vi "Main.vi"() -> ()   [LabVIEW 2015] (continued)
  out "Sigma":dbl[](array[numeric])
  out "Last Zernike":dbl[](array[numeric])
  in  "Stop AO Algorithm":bool
  in  "Step Size":dbl=0.05
  out "Metric Value":dbl(graph)=0.00227571952127783
  out "Optimal Zernike":dbl[](array[numeric])
  out "Quadratic Calc":bool
  out "Optimal Z Idx":i32
  in  "Note":string="Cou6_200x200_5mW_1580nm_step0.01"
  # "Up"
  # "Right"
  # "Left"
  # "Down"
  # "Standard Lifetimes (s):\nCoumarin 6 MeOH - 2.3E-9\nCoumarin 6 EtOH - 2.41E-9\nFluorescein NaOH - 4.0E-9\nRhodamine B H2O - 1.7E-9"
  # "V_IF (0 or -2pi)"
  # "(Shutter On)"
  # "(Shutter Off)"
  # "V_IF (0.5pi or -1.5pi)"
  # "V_IF (pi or -pi)"
  # "V_IF (1.5pi or -0.5pi)"
  # "Pixel width calibration:\n1. Move the cursor to a feature pixel that you can recognize\n2. Click \"Record X1\" to record the X coordinate\n\n \n3. Use \"X-\" or \"X+\" with \"XY Step\" of 30 um to move the image horizentally by 30 um\n4. Move the cursor to the same feature pixel\n5. Click \"Record X2\" to record the X coordinate again\n\n\n6. Click \"Pixel Width\" to calculate the pixel width (um/px)\n7. Input your desired pixel width (um/px) and the cooresponding \"XY Factor (1/V)\" will be calculated"
  # "Based on \"Desired Pixel Wdith (um)\""
  # "Going inside the sample (Z increase)"
  # "Z4\nAst45"
  # "Z5\nDef"
  # "Z6\nAst0"
  # "Z7\nTreY"
  # "Z8\nComX"
  # "Z9\nComY"
  # "Z10\nTreX"
  # "Z11\nTetY"
  # "Z12\nSAstY"
  # "Z13\nSAb3"
  # "Z14\nSAstX"
  # "Z15\nTetX"
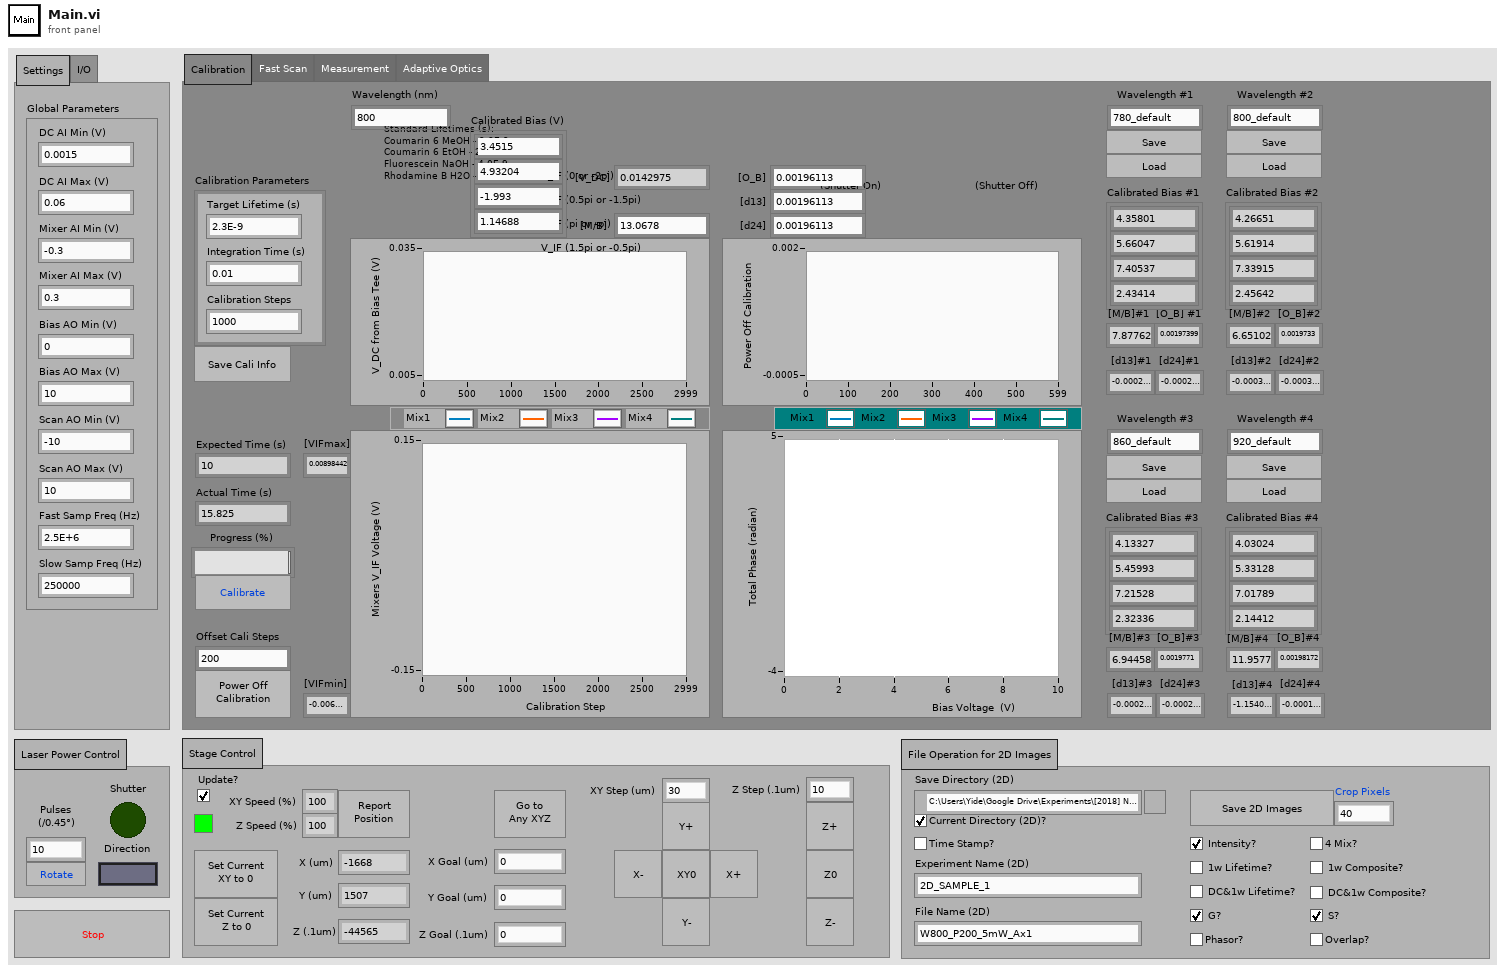
[diagram p1: front panel]
types:
  T1 = cluster{"DC AI Min (V)":dbl, "DC AI Max (V)":dbl, "Mixer AI Min (V)":dbl, "Mixer AI Max (V)":dbl, "Bias AO Min (V)":dbl, "Bias AO Max (V)":dbl, "Scan AO Min (V)":dbl, "Scan AO Max (V)":dbl, "Fast Samp Freq (Hz)":dbl, "Slow Samp Freq (Hz)":dbl}
  T2 = enum32{"Calibration", "Fast Scan", "Measurement", "Adaptive Optics"}
  T3 = cluster{"Target Lifetime (s)":dbl, "Integration Time (s)":dbl, "Calibration Steps":dbl}
  T4 = cluster{"Pixel Dwell Time (s)":dbl, "Pixel Size":dbl, "X Min (V)":dbl, "X Max (V)":dbl, "Y Min (V)":dbl, "Y Max (V)":dbl, "XY Factor (1/V)":dbl}
  T5 = enum16{"Nikon 40X NA 0.8 WD=3.5mm", "Olympus 25X NA 1.05 WD=2mm"}
  T6 = enum32{"Process", "Results", "Phasors", "Z-Stack", "Time-Lapse", "GSOS Process", "GSOS Results"}
  T7 = cluster{"X Values":dbl[], "Histogram: h(x)":i32[]}
  T8 = enum16{"fire", "rainbow", "gray", "inverse gray", "ice", "original"}
  T9 = cluster{bool[], dbl[], cluster{dbl, dbl}[], u32[]}
  T10 = enum16{"Intensity 3D", "1w Lifetime 3D", "DC&1w Lifetime 3D", "1w Composite 3D", "DC&1w Composite 3D", "Phasor 3D", "Overlap 3D"}
  T11 = enum16{"Mean Pixel Value", "Normalized Variance", "Mean Squared Pixel Value"}
  T12 = cluster{"Mixer AI Channel(s)":tag, "DC AI Channel(s)":tag, "Bias AO Channel(s) ":tag, "Scan AO Channel(s)":tag}
  T13 = enum32{"Calibration", "Fast Scan", "Measurement"}
  T14 = cluster{"DC AI task out":refnum<k21>, "Mixer AI task out":refnum<k21>, "Bias AO task out":refnum<k21>, "Scan AO task out":refnum<k21>}
  T15 = typedef "NI_LVConfig.lvlib/Config Data RefNum.ctl" = refnum<k1>
  T16 = typedef "LVBoundsTypeDef.ctl" = cluster{"Width":u32, "Height":u32}
  T17 = typedef "lveventtype.ctl" = enum32{"Null", "Timeout", "Annotation Menu Selection", "Annotation Menu Selection?", "App Instance Close", "App Instance Close?", "Autoscale Range Change", "Bookmark Info Change", "Cell Edit", "Cell Edit?", "Cursor Grab", "Cursor Grab?", "Cursor Menu Selection", "Cursor Menu Selection?", "Cursor Move", "Cursor Release", "Data Change", "Direction Change", "Display State Change", "Drag Ended", "Drag Enter", "Drag Leave", "Drag Over", "Drag Source Update", "Drag Starting", "Drag Starting?", "Drop", "Exec State Change", "Key Down", "Key Down?", "Key Repeat", "Key Repeat?", "Key Up", "Listbox Double Click", "Menu Activation?", "Menu Selection (App)", "Menu Selection? (App)", "Menu Selection (User)", "Mouse Down", "Mouse Down?", "Mouse Enter", "Mouse Leave", "Mouse Move", "Mouse Up", "Mouse Wheel", "NI Security User Change (App)", "Pane Size", "Panel Close", "Panel Close?", "Panel Resize", "Plot Attribute Change", "Scale Range Change", "Shortcut Menu Activation?", "Shortcut Menu Selection (App)", "Shortcut Menu Selection? (App)", "Shortcut Menu Selection (User)", "Tree Double Click", "Tree Drag", "Tree Drag?", "Tree Drop", "Tree Drop?", "Tree Item Close", "Tree Item Close?", "Tree Item Open", "Tree Item Open?", "User Event", "Value Change"}
  T18 = typedef "LVRectTypeDef.ctl" = cluster{"Left":i16, "Top":i16, "Right":i16, "Bottom":i16}
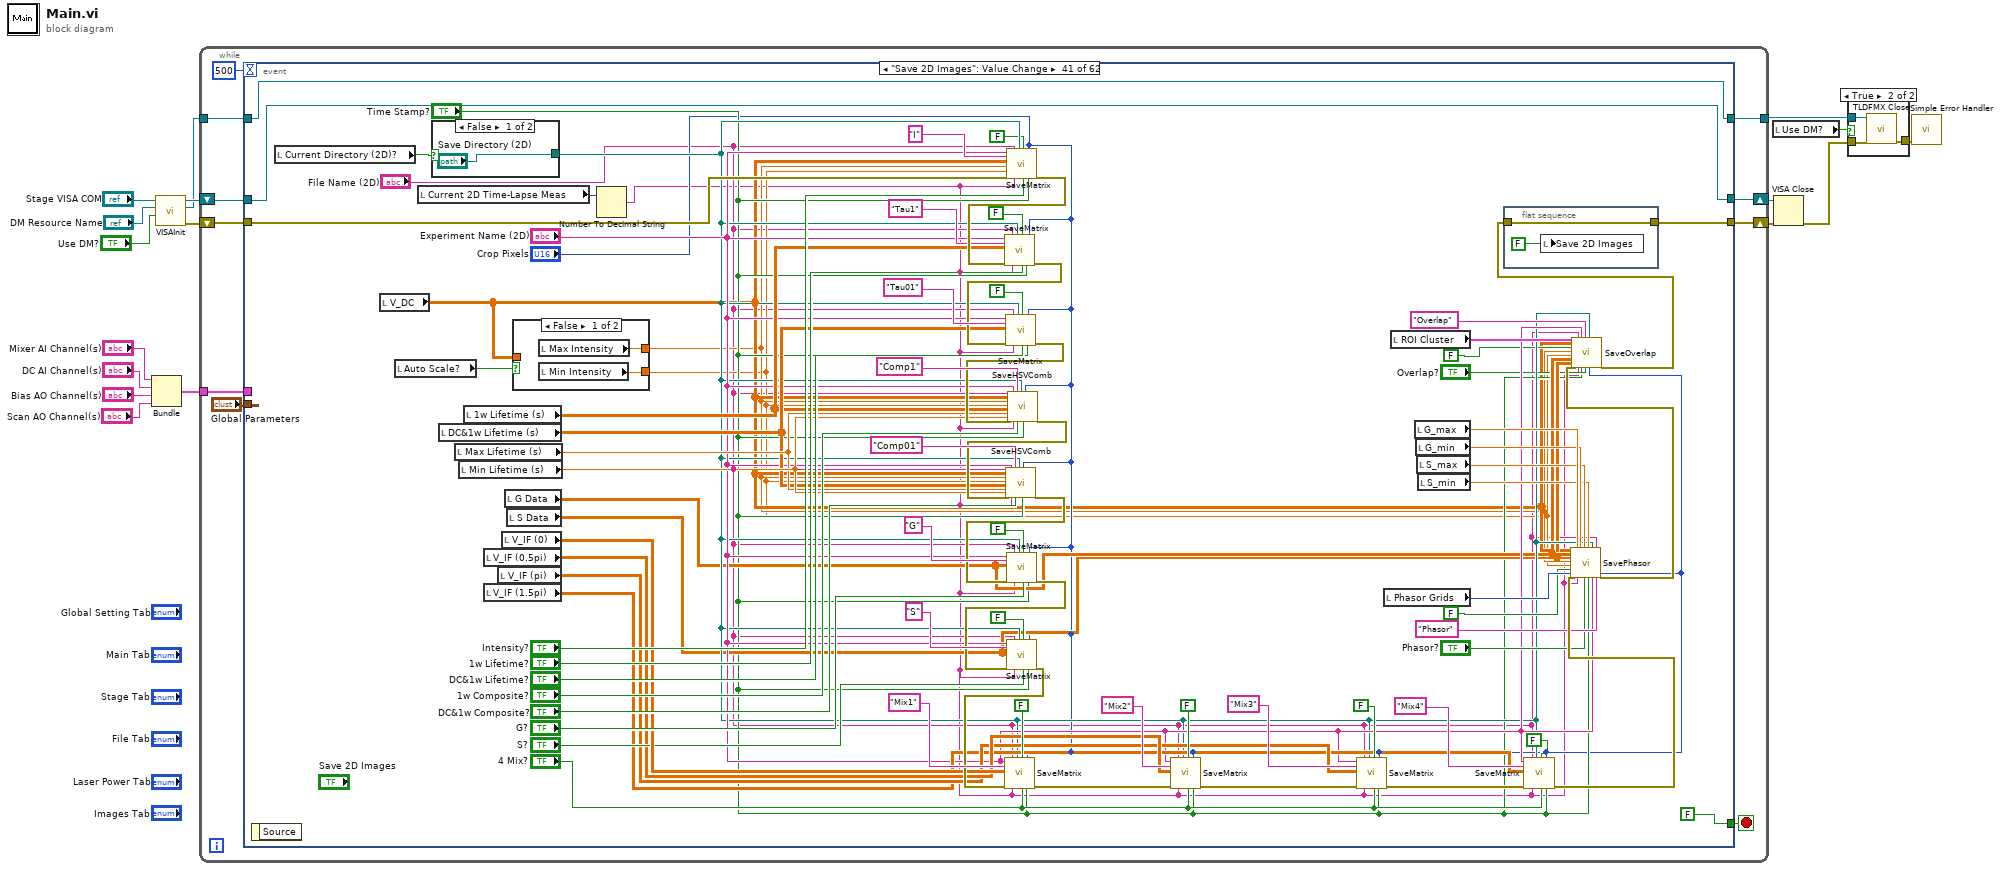
[diagram p0: block diagram]
diagram:
  n1 = Bundle("Mixer AI Channel(s)"="Mixer AI Channel(s)", "DC AI Channel(s)"="DC AI Channel(s)", "Bias AO Channel(s)"="Bias AO Channel(s)", "Scan AO Channel(s)"="Scan AO Channel(s)") -> (w13:T12)  [unwired: 1 in]
  n2 = call "VISAInit.vi"("Use DM?"="Use DM?", "DM Resource Name"="DM Resource Name", "Stage Resource Name"="Stage VISA COM") -> ("error out"=w12:errorcluster, "DM Handle"=w8:refnum<visa-resource-name>, "Stage Resource"=w11:refnum<visa-resource-name>)  [unwired: 6 in]
  n3 = while {
    shift-right: [w22] -> w17
    shift-left: w11 -> [w27]
    shift-right: [w21] -> w16
    shift-left: w12 -> [w26]
    tunnel: w13 -> [w25]
    tunnel: w8 -> [w20]
    tunnel: [w19] -> w5
    stop <- w24 stop-if-true
    n4 = event shown="[40] \"Save 2D Images\": Value Change" {
      selector: _ -> [_ _ _ _ _ _ _ _ _ _ _ _ _ _ _ _ _ _ _ _ _ _ _ _ _ _ _ _ _ _ _ _ _ _ _ _ _ _ _ _ _ _ _ _ _ _ _ _ _ _ _ _ _ _ _ _ _ _ _ _ _ _]
      dyn-events: _ -> [_ _ _ _ _ _ _ _ _ _ _ _ _ _ _ _ _ _ _ _ _ _ _ _ _ _ _ _ _ _ _ _ _ _ _ _ _ _ _ _ _ _ _ _ _ _ _ _ _ _ _ _ _ _ _ _ _ _ _ _ _ _]
      timeout: 500 -> [_ _ _ _ _ _ _ _ _ _ _ _ _ _ _ _ _ _ _ _ _ _ _ _ _ _ _ _ _ _ _ _ _ _ _ _ _ _ _ _ _ _ _ _ _ _ _ _ _ _ _ _ _ _ _ _ _ _ _ _ _ _]
      tunnel: [FALSE ("Shutter") FALSE ("Shutter") FALSE ("Shutter") FALSE ("Shutter") FALSE ("Shutter") FALSE ("Shutter") FALSE ("Shutter") FALSE ("Shutter") FALSE ("Shutter") FALSE ("Shutter") FALSE ("Shutter") FALSE ("Shutter") FALSE ("Shutter") FALSE ("Shutter") FALSE ("Shutter") _ FALSE ("Shutter") _ _ _ _ FALSE ("Shutter") _ FALSE ("Shutter") FALSE ("Shutter") FALSE ("Shutter") FALSE ("Shutter") FALSE ("Shutter") FALSE ("Shutter") FALSE ("Shutter") FALSE ("Shutter") FALSE ("Shutter") FALSE ("Shutter") FALSE ("Shutter") FALSE ("Shutter") FALSE ("Shutter") FALSE ("Shutter") FALSE ("Shutter") FALSE ("Shutter") FALSE ("Shutter") FALSE ("Shutter") FALSE ("Shutter") FALSE ("Shutter") FALSE ("Shutter") "Stop" FALSE ("Shutter") FALSE ("Shutter") FALSE ("Shutter") FALSE ("Shutter") FALSE ("Shutter") FALSE ("Shutter") FALSE ("Shutter") FALSE ("Shutter") FALSE ("Shutter") FALSE ("Shutter") FALSE ("Shutter") FALSE ("Shutter") FALSE ("Shutter") FALSE ("Shutter") FALSE ("Shutter") FALSE ("Shutter") FALSE ("Shutter")] -> w24
      tunnel: w27 -> [w33 w89 w118 w274 w360 w382 w392 w402 w410 w422 w432 w442 w452 w469 w567 w585 w592 w630 w644 w681 w799 w886 w959 w1094 w1262 w1335 w1456 w1614 w1638 w1677 w1744 w1785 w1814 w1978 w2043 w2086 w2134 w2189 w2276 w2330 w2439 w2454 w2462 w2469 w2479 w2498 w2516 w2534 w2552 w2554 w2572 w2600 w2610 w2631 w2640 w2652 w2684 w2704 w2708 w2720 w2726 w2745]
      tunnel: w26 -> [w34 w87 w117 w271 w361 w381 w391 w401 w409 w421 w431 w441 w451 w461 w554 w582 w599 w626 w638 w677 w798 w881 w955 w1083 w1259 w1334 w1432 w1608 w1629 w1668 w1708 w1752 w1844 w1969 w2040 w2060 w2110 w2164 w2277 w2343 w2392 w2453 w2461 w2468 w2478 w2497 w2515 w2533 w2551 w2553 w2571 w2599 w2609 w2630 w2639 w2651 w2685 w2702 w2710 w2719 w2725 w2744]
      tunnel: [w29 w89 w116 w273 w360 w382 w392 w402 w410 w422 w432 w442 w452 w468 w567 w585 w592 w630 w644 w681 w799 w886 w959 w1079 w1261 w1321 w1456 w1614 w1638 w1677 w1744 w1785 w1814 w1978 w2043 w2086 w2134 w2189 w2276 w2330 w2439 w2454 w2462 w2469 w2479 w2486 w2503 w2520 w2539 w2558 w2576 w2594 w2605 w2616 w2636 w2648 w2661 w2704 w2708 w2720 w2726 w2745] -> w22
      tunnel: [w28 w86 w110 w270 w338 w381 w391 w401 w409 w421 w431 w441 w451 w459 w557 w580 w593 w624 w640 w683 w795 w876 w958 w1085 w1258 w1319 w1446 w1586 w1628 w1667 w1710 w1751 w1822 w1946 w2039 w2049 w2098 w2153 w2245 w2331 w2410 w2453 w2460 w2467 w2477 w2485 w2502 w2521 w2538 w2559 w2577 w2593 w2606 w2617 w2637 w2649 w2660 w2701 w2709 w2719 w2725 w2744] -> w21
      tunnel: w25 -> [_ _ w114 w269 _ _ _ _ _ _ _ _ _ w467 _ _ _ _ _ _ _ _ _ w1088 _ _ _ _ _ _ _ _ _ _ _ _ _ _ _ _ _ _ _ _ _ _ _ _ _ _ _ _ _ _ _ _ _ _ _ _ _ _]
      tunnel: "Global Parameters" -> [_ _ w112 w268 _ _ _ _ _ _ _ _ _ w466 _ _ _ _ _ _ _ _ _ w1086 _ _ _ _ _ _ _ _ _ _ _ _ _ _ _ _ _ _ _ _ _ _ _ _ _ _ _ _ _ _ _ _ _ _ _ _ _ _]
      tunnel: [w32 w80 w96 w266 w327 w379 w386 w396 w406 w416 w426 w436 w446 w458 w558 w581 w591 w629 w645 w679 w796 w879 w957 w1073 w1257 w1318 w1420 w1585 w1627 w1666 w1703 w1748 w1789 w1933 w2024 w2045 w2093 w2141 w2196 w2309 w2361 w2451 w2458 w2464 w2470 w2482 w2500 w2518 w2536 w2556 w2574 w2590 w2602 w2614 w2634 w2646 w2658 w2700 w2706 w2712 w2722 w2732] -> w19
      tunnel: w20 -> [w32 w80 w96 w266 w327 w379 w386 w396 w406 w416 w426 w436 w446 w458 w555 w583 w597 w629 w645 w680 w797 w880 w956 w1073 w1257 w1318 w1420 w1585 w1627 w1666 w1703 w1748 w1789 w1933 w2024 w2045 w2093 w2141 w2196 w2309 w2361 w2451 w2458 w2464 w2470 w2482 w2500 w2518 w2536 w2556 w2574 w2590 w2602 w2614 w2634 w2646 w2658 w2700 w2706 w2712 w2722 w2732]
      event Timeout {
        n5 = event-data() -> ()  [unwired: 1 in, 1 out]
        n6 = case shown="True" "Update?" {
          tunnel: w34 -> [w35 w62]
          tunnel: w33 -> [w36 w61]
          tunnel: [w36 w37] -> w29
          tunnel: [w35 w38] -> w28
          frame False {
          }
          frame True {
            n7 = local read "Timeout Indicator"() -> (w42:bool)
            n8 = VISA Write(VISA resource name=w61, write buffer="P" ("string"), error in (no error)=w62) -> (VISA resource name out=w70:refnum<visa-resource-name>, error out=w69:errorcluster)  [unwired: 1 out]
            n9 = Not(x=w42) -> (.not. x?=→"Timeout Indicator":bool)
            n10 = VISA Read(VISA resource name=w70, byte count=u32 256, error in (no error)=w69) -> (VISA resource name out=w48:refnum<visa-resource-name>, read buffer=w75:string, error out=w50:errorcluster)  [unwired: 1 out]
            n11 = Search/Split String(string=w75, search string/char (-)=",") -> (substring before match=→"X (um)":string, match + rest of string=w67:string)  [unwired: 1 in, 1 out]
            n12 = Search/Split String(string=w67, search string/char (-)=",", offset (0)=1) -> (substring before match=w64:string, match + rest of string=w77:string)  [unwired: 1 out]
            n13 = VISA Clear(VISA resource name=w48, error in (no error)=w50) -> (VISA resource name out=w47:refnum<visa-resource-name>, error out=w49:errorcluster)
            n14 = String Subset(string=w64, offset (0)=1) -> (substring=→"Y (um)":string)  [unwired: 1 in]
            n15 = String Subset(string=w77, offset (0)=1) -> (substring=→"Z (.1um)":string)  [unwired: 1 in]
            n16 = VISA Write(VISA resource name=w47, write buffer="O" ("string"), error in (no error)=w49) -> (VISA resource name out=w58:refnum<visa-resource-name>, error out=w59:errorcluster)  [unwired: 1 out]
            n17 = VISA Read(VISA resource name=w58, byte count=u32 256, error in (no error)=w59) -> (VISA resource name out=w46:refnum<visa-resource-name>, read buffer=→"XY Speed (%)":string, error out=w45:errorcluster)  [unwired: 1 out]
            n18 = VISA Clear(VISA resource name=w46, error in (no error)=w45) -> (VISA resource name out=w44:refnum<visa-resource-name>, error out=w43:errorcluster)
            n19 = VISA Write(VISA resource name=w44, write buffer="OF" ("string"), error in (no error)=w43) -> (VISA resource name out=w53:refnum<visa-resource-name>, error out=w54:errorcluster)  [unwired: 1 out]
            n20 = VISA Read(VISA resource name=w53, byte count=u32 256, error in (no error)=w54) -> (VISA resource name out=w40:refnum<visa-resource-name>, read buffer=→"Z Speed (%)":string, error out=w39:errorcluster)  [unwired: 1 out]
            n21 = VISA Clear(VISA resource name=w40, error in (no error)=w39) -> (VISA resource name out=w37:refnum<visa-resource-name>, error out=w38:errorcluster)
          }
        }
      }
      event Panel Close? {
        n22 = event-data() -> ()  [unwired: 1 in, 1 out]
        n23 = call "ShutterControl.vi"("error in"=w87, "Shutter"=FALSE) -> ("error out"=w86:errorcluster, "Status Indicator"=w85:bool)  [unwired: 8 in]
        n24 = local write "Shutter"(w85) -> ()
        n25 = Two Button Dialog(message="Do you really want to exit?") -> (T button?=w91:bool)  [unwired: 2 in]
        n26 = local write "Meas Progress"(0.0 ("Fast Scan Progress")) -> ()
        n27 = local write "Fast Scan Progress"(0.0 ("Fast Scan Progress")) -> ()
        n28 = local write "Measure"(FALSE ("Fast Scan")) -> ()
        n29 = local write "Fast Scan"(FALSE ("Fast Scan")) -> ()
        n30 = Not(x=w91) -> (.not. x?=w90:bool)
        n31 = event-data("Discard?"=w90) -> ()  [unwired: 1 in, 1 out]
      }
      event "Calibrate": Value Change {
        n32 = event-data() -> ()  [unwired: 1 in, 1 out]
        n33 = flat-sequence {
          tunnel: w118 -> [w127]
          tunnel: [w127] -> w122
          tunnel: [w126] -> w121
          tunnel: w117 -> [w126]
          tunnel: [w125] -> w120
          tunnel: [w124] -> w115
          tunnel: w114 -> [w124]
          tunnel: w112 -> [w123]
          tunnel: [w123] -> w113
          tunnel: w122 -> [w183]
          tunnel: [w183] -> w119
          tunnel: w121 -> [w182]
          tunnel: w120 -> [w145]
          tunnel: w115 -> [w154]
          tunnel: w113 -> [w174]
          tunnel: [w155] -> w111
          tunnel: [w174] -> w109
          tunnel: ["Calibration Parameters"] -> w108
          tunnel: [w172] -> w107
          tunnel: [w171] -> w106
          tunnel: [w168] -> w105
          tunnel: [w167] -> w104
          tunnel: [w166] -> w103
          tunnel: [w162] -> w102
          tunnel: [w146] -> w101
          tunnel: [w145] -> w98
          tunnel: [w133] -> w94
          tunnel: [w132] -> w93
          tunnel: w119 -> [w251]
          tunnel: w111 -> [w250]
          tunnel: w109 -> [w249]
          tunnel: w108 -> [w248]
          tunnel: w107 -> [w244]
          tunnel: w106 -> [w243]
          tunnel: w105 -> [w242]
          tunnel: w104 -> [w241]
          tunnel: w103 -> [w240]
          tunnel: w102 -> [w238]
          tunnel: w101 -> [w233]
          tunnel: [w251] -> w100
          tunnel: [w250] -> w99
          tunnel: w98 -> [w234]
          tunnel: [w234] -> w97
          tunnel: w94 -> [w231]
          tunnel: w93 -> [w230]
          tunnel: [w261] -> w110
          tunnel: [w262] -> w116
          tunnel: w100 -> [w262]
          tunnel: w99 -> [w261]
          tunnel: w97 -> [w255]
          frame #0 {
            n34 = Tick Count (ms)() -> (millisecond timer value=w125:u32)
          }
          frame #1 {
            w136 = 0.0
            w180 = T13."Calibration" ("Main Tab")
            n35 = flat-sequence {
              tunnel: [w192] -> w143
              tunnel: w147 -> [w192]
              frame #0 {
                n36 = Wait (ms)(milliseconds to wait=u32 100) -> ()  [unwired: 1 out]
              }
            }
            n37 = call "DAQInit.vi"("Calibration Parameters"="Calibration Parameters", "error in"=w182, "Functions"=w180, "Global Parameters"=w174, "DAQ Channels"=w154) -> ("error out"=w176:errorcluster, "Expected Time (s)"=→"Expected Time (s)":dbl, "Tasks Out"=w153:T14)  [unwired: 4 in]
            n38 = Unbundle By Name("Calibration Parameters") -> ("Calibration Steps"=w179:dbl)
            n39 = call "ShutterControl.vi"("error in"=w176, "Shutter"=TRUE) -> ("error out"=w158:errorcluster, "Status Indicator"=w170:bool)  [unwired: 8 in]
            n40 = local write "Shutter"(w170) -> ()
            n41 = flat-sequence {
              tunnel: [w198] -> w157
              tunnel: w158 -> [w198]
              frame #0 {
                n42 = Wait (ms)(milliseconds to wait=u32 100) -> ()  [unwired: 1 out]
              }
            }
            n43 = while {
              tunnel: w153 -> [w225]
              tunnel: w157 -> [w224]
              tunnel: w180 -> [w208]
              tunnel: "Calibration Parameters" -> [w222]
              tunnel: w174 -> [w220]
              tunnel: w179 -> [w221]
              tunnel: [w214] -> w171 mode=concatenating
              tunnel: [w217] -> w156
              tunnel: [w219] -> w144
              tunnel: [w208] -> w178
              tunnel: [w209] -> w172 mode=indexing
              tunnel: [w212] -> w168 mode=concatenating
              tunnel: [w211] -> w167 mode=concatenating
              tunnel: [w210] -> w166 mode=concatenating
              tunnel: [w207] -> w159 mode=concatenating
              i -> [w229]
              stop <- w215 stop-if-true
              n44 = To Double Precision Float(number=w229) -> (double precision float=w203:dbl)
              n45 = call "ImageFrame.vi"("Tasks In"=w225, "Global Parameters"=w220, "Calibration Parameters"=w222, "Functions"=w208, "error in"=w224, "index"=w203) -> ("Tasks Out"=w219:T14, "Mixer AI Channels Data"=w206:dbl[][], "DC AI Channel Date"=w205:dbl[], "Bias Voltage"=w209:dbl, "error out"=w217:errorcluster)  [unwired: 5 in]
              n46 = Increment(x=w203) -> (x+1=w204:dbl)
              n47 = call "Analysis.vi"("Functions"=w208, "DC AI Channel Data"=w205, "Mixer AI Channels Data"=w206) -> ("AI Mix4 Data"=w210:dbl[], "AI Mix3 Data"=w211:dbl[], "AI Mix2 Data"=w212:dbl[], "AI Mix1 Data"=w214:dbl[], "AI DC Data"=w207:dbl[])  [unwired: 3 in, 1 out]
              "Calibration AI  Signals (Integrated) 2" <- w207
              n48 = Unbundle By Name(w217) -> ("status"=w218:bool)
              n49 = Greater Or Equal?(x=w204, y=w221) -> (x >= y?=w216:bool)
              n50 = Divide(x=w204, y=w221) -> (x/y=w228:dbl)
              n51 = Build Array(w214, w212, w211, w210) -> (→"Calibration AI  Signals (Integrated)":dbl[][])
              n52 = Multiply(x=w228, y=100.0) -> (x*y=w226:dbl)
              n53 = Compound Arithmetic op=OR(w218, w216) -> (w215:bool)
              n54 = To Unsigned Byte Integer(number=w226) -> (unsigned 8bit integer=→"Calibrate Progress":u8)
            }
            n55 = call "PowerOffCalibration.vi"("Tasks In"=w144, "Offset Cali Steps"="Offset Cali Steps", "error in"=w143) -> ("Tasks Out"=w141:T14, "V_DC Array"=w131:dbl[], "d13 Array"=w130:dbl[], "d24 Array"=w129:dbl[], "error out"=w140:errorcluster)  [unwired: 8 in]
            n56 = Build Array(w131, w130, w129) -> (→"Power Off Voltages":dbl[][])
            n57 = call "ShutterControl.vi"("error in"=w156, "Shutter"=FALSE) -> ("error out"=w147:errorcluster, "Status Indicator"=w169:bool)  [unwired: 8 in]
            n58 = local write "Shutter"(w169) -> ()
            n59 = for {
              tunnel: w131 -> [w196] mode=indexing
              shift-right: [w194] -> w148
              shift-left: 0.0 -> [w195]
              tunnel: [w193] -> w151
              i -> [w193]
              n60 = Add(x=w196, y=w195) -> (x+y=w194:dbl)
            }
            n61 = for {
              tunnel: w159 -> [w202] mode=indexing
              shift-right: [w200] -> w165
              shift-left: 0.0 -> [w201]
              tunnel: [w199] -> w161
              i -> [w199]
              n62 = Add(x=w202, y=w201) -> (x+y=w200:dbl)
            }
            n63 = for {
              tunnel: w130 -> [w190] mode=indexing
              shift-right: [w188] -> w139
              shift-left: w136 -> [w189]
              tunnel: [w187] -> w137
              tunnel: w129 -> [w186] mode=indexing
              shift-right: [w184] -> w135
              shift-left: w136 -> [w185]
              i -> [w187]
              n64 = Add(x=w190, y=w189) -> (x+y=w188:dbl)
              n65 = Add(x=w186, y=w185) -> (x+y=w184:dbl)
            }
            n66 = Increment(x=w137) -> (x+1=w138:i32)
            n67 = Increment(x=w151) -> (x+1=w152:i32)
            n68 = Increment(x=w161) -> (x+1=w160:i32)
            n69 = To Double Precision Float(number=w138) -> (double precision float=w134:dbl)
            n70 = To Double Precision Float(number=w152) -> (double precision float=w149:dbl)
            n71 = To Double Precision Float(number=w160) -> (double precision float=w164:dbl)
            n72 = Divide(x=w139, y=w134) -> (x/y=w133:dbl)
            n73 = Divide(x=w148, y=w149) -> (x/y=w146:dbl)
            n74 = Divide(x=w135, y=w134) -> (x/y=w132:dbl)
            n75 = Divide(x=w165, y=w164) -> (x/y=w162:dbl)
            n76 = call "DAQClose.vi"("error in"=w140, "Functions"=w178, "Tasks In"=w141, "DAQ Channels"=w154) -> ("error out"=w155:errorcluster)  [unwired: 7 in]
          }
          frame #2 {
            n77 = local write "[d13]"(w231) -> ()
            n78 = local write "[d24]"(w230) -> ()
            n79 = call "PhaseCalibration.vi"("Global Parameters"=w249, "Bias Voltages"=w244, "Calibration Parameters"=w248, "Mixer1 Values"=w243, "Mixer2 Values"=w242, "Mixer3 Values"=w241, "Mixer4 Values"=w240, "[V_DC]"=w238, "[O_B]"=w233) -> ("Mixer Phases"=→"Mixer Phases":cluster{"Bias voltage":dbl[], dbl[]}[], "Calibrated Bias Voltages"=w237:dbl[], "[M/B]"=w232:dbl, "[V_IF_max]"=→"[VIFmax]":dbl, "[V_IF_min]"=→"[VIFmin]":dbl)  [unwired: 2 in]
            n80 = local write "[O_B]"(w233) -> ()
            n81 = Greater?(x=w237, y=10.0) -> (0:w246:bool[])
            n82 = local write "[M/B]"(w232) -> ()
            n83 = Or Array Elements(Boolean array=w246) -> (logical OR=w245:bool)
            n84 = case shown="False" w245 {
              tunnel: w237 -> [w252 _]
              frame False {
                n85 = local write "Calibrated Bias (V)"(w252) -> ()
              }
              frame True {
                n86 = One Button Dialog(message="Calibration failed.\nVoltage out of bound.\nPlease re-calibrate.") -> ()  [unwired: 1 in, 1 out]
              }
            }
            "[V_DC]" <- w238
          }
          frame #3 {
            n87 = Tick Count (ms)() -> (millisecond timer value=w257:u32)
            n88 = Subtract(x=w257, y=w255) -> (x-y=w258:u32)
            n89 = local write "Calibrate"(FALSE ("Fast Scan")) -> ()
            n90 = To Double Precision Float(number=w258) -> (double precision float=w259:dbl)
            n91 = Divide(x=w259, y=1000.0) -> (x/y=→"Actual Time (s)":dbl)
          }
        }
      }
      event "PowerOffCalibration": Value Change {
        n92 = event-data() -> ()  [unwired: 1 in, 1 out]
        n93 = flat-sequence {
          tunnel: [w308] -> w275
          tunnel: w274 -> [w308]
          tunnel: [w293] -> w272
          tunnel: w271 -> [w305]
          tunnel: w269 -> [w295]
          tunnel: w268 -> [w303]
          tunnel: [w296] -> w267
          tunnel: [w281] -> w264
          tunnel: [w280] -> w263
          tunnel: w275 -> [w325]
          tunnel: [w325] -> w273
          tunnel: w272 -> [w324]
          tunnel: [w324] -> w270
          tunnel: w267 -> [w323]
          tunnel: w264 -> [w321]
          tunnel: w263 -> [w320]
          frame #0 {
            w284 = 0.0
            w294 = T13."Calibration" ("Main Tab")
            n94 = local read "Calibration Parameters"() -> (w302:T3)
            n95 = call "DAQInit.vi"("Calibration Parameters"=w302, "error in"=w305, "Functions"=w294, "Global Parameters"=w303, "DAQ Channels"=w295) -> ("error out"=w304:errorcluster, "Tasks Out"=w291:T14)  [unwired: 4 in, 1 out]
            n96 = call "ShutterControl.vi"("error in"=w304, "Shutter"=FALSE) -> ("error out"=w292:errorcluster, "Status Indicator"=w306:bool)  [unwired: 8 in]
            n97 = local write "Shutter"(w306) -> ()
            n98 = local read "Offset Cali Steps"() -> (w290:dbl)
            n99 = call "PowerOffCalibration.vi"("Tasks In"=w291, "Offset Cali Steps"=w290, "error in"=w292) -> ("Tasks Out"=w289:T14, "V_DC Array"=w278:dbl[], "d13 Array"=w277:dbl[], "d24 Array"=w276:dbl[], "error out"=w288:errorcluster)  [unwired: 8 in]
            n100 = Build Array(w278, w277, w276) -> (w279:dbl[][])
            n101 = local write "Power Off Voltages"(w279) -> ()
            n102 = for {
              tunnel: w278 -> [w319] mode=indexing
              shift-right: [w317] -> w297
              shift-left: 0.0 -> [w318]
              tunnel: [w316] -> w300
              i -> [w316]
              n103 = Add(x=w319, y=w318) -> (x+y=w317:dbl)
            }
            n104 = for {
              tunnel: w277 -> [w315] mode=indexing
              shift-right: [w313] -> w287
              shift-left: w284 -> [w314]
              tunnel: [w312] -> w285
              tunnel: w276 -> [w311] mode=indexing
              shift-right: [w309] -> w283
              shift-left: w284 -> [w310]
              i -> [w312]
              n105 = Add(x=w315, y=w314) -> (x+y=w313:dbl)
              n106 = Add(x=w311, y=w310) -> (x+y=w309:dbl)
            }
            n107 = Increment(x=w285) -> (x+1=w286:i32)
            n108 = Increment(x=w300) -> (x+1=w301:i32)
            n109 = call "DAQClose.vi"("error in"=w288, "Functions"=w294, "Tasks In"=w289, "DAQ Channels"=w295) -> ("error out"=w293:errorcluster)  [unwired: 7 in]
            n110 = To Double Precision Float(number=w286) -> (double precision float=w282:dbl)
            n111 = To Double Precision Float(number=w301) -> (double precision float=w298:dbl)
            n112 = Divide(x=w287, y=w282) -> (x/y=w281:dbl)
            n113 = Divide(x=w283, y=w282) -> (x/y=w280:dbl)
            n114 = Divide(x=w297, y=w298) -> (x/y=w296:dbl)
          }
          frame #1 {
            n115 = local write "[O_B]"(w323) -> ()
            n116 = local write "[d13]"(w321) -> ()
            n117 = local write "[d24]"(w320) -> ()
            n118 = local write "PowerOffCalibration"(FALSE ("Re-Calibrate O")) -> ()
          }
        }
      }
      event "Save Calibration Info": Value Change {
        w332 = "Calibration" ("string")
        n119 = event-data() -> ()  [unwired: 1 in, 1 out]
        n120 = Current VI's Path() -> (path=w359:path)
        n121 = Strip Path(path=w359) -> (stripped path=w362:path)  [unwired: 1 out]
        n122 = local read "Mixer Phases"() -> (w337:cluster{"X":dbl[], "Y":dbl[]}[])
        n123 = Concatenate Strings(w332, "_" ("string"), "Wavelength (nm)", "nm" ("string")) -> (w329:string)
        n124 = Build Path(base path=w362, name or relative path=w332) -> (appended path=w363:path)